vi "UHR-Fleezers Control (host) - 12.8.vi"() -> ()   [LabVIEW 2012] (continued)
        "Time/f+b scan (s) (MCL)" <- w1868
        n1295 = Divide(x=w1894, y=w1874) -> (x/y=→"N sets should be saved (MCL)":dbl)
        n1296 = Multiply(x=w1868, y=w1867) -> (x*y=→"Total Time (s)":dbl)
        n1297 = Not(x="Fast Scan Dir") -> (.not. x?=w1872:bool)
        n1298 = xnode "Read/Write Control"("FPGA VI Reference In"=w1860, "Scan steps (MCL)"="Scan steps (MCL)", "Number of scans (MCL)"=w1867, "Cycles per step (MCL)"=w1885, "Scan freq.  increment (MCL)"=w1865, "1D or 2D Scan?"="2D or 1D Scan", "MCL Scan Axis"=w1872, "Cont. Scan (MCL)"="Continuous MCL Scanning") -> ("error out"=w1896:errorcluster)  [unwired: 1 in, 1 out]
      }
      event "Read Cal": Value Change {
        w1898 = 1000.0 ("y")
        n1299 = event-data() -> ()  [unwired: 7 out]
        n1300 = local read "Save file name"() -> (w1923:path)
        n1301 = local write "Read Cal"(FALSE ("Read Cal")) -> ()
        n1302 = Strip Path(path=w1923) -> (stripped path=w1922:path)  [unwired: 1 out]
        n1303 = Path To String(path=w1922) -> (string=w1921:string)
        n1304 = Concatenate Strings(w1921, "\\current.cal" ("string")) -> (w1919:string)
        n1305 = String To Path(string=w1919) -> (path=w1918:path)
        n1306 = Open/Create/Replace File(file path (use dialog)=w1918, operation (0:open)=T29."open", access (0:read/write)=enum16{"read/write", "read-only", "write-only"}."read-only") -> (refnum out=w1926:refnum<file>, error out=w1912:errorcluster)  [unwired: 1 in, 3 out]
        n1307 = Deny Access(4:w1912, 7:w1926) -> (0:w1911:errorcluster, 3:w1917:refnum<file>)  [unwired: 1 out]
        n1308 = Read from Binary File(5:0.0, 8:w1911, 9:T28."big-endian, network order" ("byte order (0:big-endian, network order)"), 10:-1 ("count (1)"), 11:w1917) -> (0:w1910:errorcluster, 2:w1908:dbl[], 3:w1913:refnum<file>)  [unwired: 2 out]
        n1309 = Array To Cluster(array=w1908) -> (cluster=w1907:T31)
        n1310 = Unbundle(w1907) -> ("[0]"=w1906:dbl, "[1]"=w1905:dbl, "[2]"=w1904:dbl, "[3]"=w1903:dbl, "[4]"=w1902:dbl, "[5]"=w1901:dbl)
        n1311 = Close File(refnum=w1913, error in=w1910) -> (error out=→"Read cal error":errorcluster)  [unwired: 1 out]
        n1312 = Multiply(x=w1901, y=w1898) -> (x*y=w1899:dbl)
        n1313 = local write "T2 kappa_x (pN/nm)"(w1903) -> ()
        n1314 = local write "T1 kappa_x (pN/nm)"(w1904) -> ()
        n1315 = local write "T1 alpha_x (nm/V)"(w1906) -> ()
        n1316 = local write "T2 alpha_x (nm/V)"(w1905) -> ()
        n1317 = Multiply(x=w1902, y=w1898) -> (x*y=w1900:dbl)
        n1318 = local write "T1 offset_x (mV)"(w1900) -> ()
        n1319 = local write "T2 offset_x (mV)"(w1899) -> ()
      }
      event "Abort MCL Scan": Value Change {
        n1320 = event-data() -> ()  [unwired: 7 out]
        n1321 = local write "MCL Scanning"(FALSE ("MCL Scanning")) -> ()
        n1322 = xnode "Read/Write Control"("FPGA VI Reference In"=w1927, "Abort scan (MCL)"="Abort MCL Scan") -> ("error out"=w1930:errorcluster)  [unwired: 1 in, 1 out]
      }
      event "Update Count (MCL)": Value Change {
        n1323 = event-data() -> ()  [unwired: 7 out]
        n1324 = xnode "Read/Write Control"("FPGA VI Reference In"=w1931, "MCL count"="Update Count (MCL)") -> ("error out"=w1933:errorcluster)  [unwired: 1 in, 1 out]
      }
      event "+ phase (MCL)", "- phase (MCL)": Value Change {
        n1325 = event-data() -> ()  [unwired: 7 out]
        n1326 = Or(x="- phase (MCL)", y="+ phase (MCL)") -> (x .or. y?=w1937:bool)
        n1327 = Negate(x="Phase adjust (MCL)") -> (-x=w1943:i16)
        n1328 = Select(t=w1943, s="+ phase (MCL)", f="Phase adjust (MCL)") -> (s? t:f=w1941:i16)
        n1329 = xnode "Read/Write Control"("FPGA VI Reference In"=w1934, "Phase count adjustment (MCL)"=w1941) -> ("FPGA VI Reference Out"=w1938:T20, "error out"=w1939:errorcluster)  [unwired: 1 in]
        n1330 = xnode "Read/Write Control"("FPGA VI Reference In"=w1938, "error in"=w1939, "+ phase (MCL)"=w1937) -> ("error out"=w1936:errorcluster)  [unwired: 1 out]
      }
      event "Abort AOD Scan": Value Change {
        n1331 = event-data() -> ()  [unwired: 7 out]
        n1332 = xnode "Read/Write Control"("FPGA VI Reference In"=w1944, "Abort scan"="Abort AOD Scan") -> ("error out"=w1946:errorcluster)  [unwired: 1 in, 1 out]
      }
      event "Continuous AOD Scanning": Value Change {
        n1333 = event-data() -> ()  [unwired: 7 out]
        n1334 = xnode "Read/Write Control"("FPGA VI Reference In"=w1947, "Cont. Scan"="Continuous AOD Scanning") -> ("error out"=w1949:errorcluster)  [unwired: 1 in, 1 out]
      }
      event "Index": Value Change {
        n1335 = event-data() -> ()  [unwired: 7 out]
        n1336 = call "Create new save file.vi"("Insert"="", "Ext"=".dat" ("string"), "Index In"="Index") -> ("Path Out"=→"Save file name":path, "Index Out"=w1950:dbl)
        "Save index" <- w1950
        n1337 = local write "Index"(w1950) -> ()
      }
      event "AO1", "AO2": Value Change {
        w1964 = 10.0 ("y")
        w1963 = 32767.0 ("y")
        n1338 = event-data() -> ()  [unwired: 7 out]
        n1339 = local read "AO2"() -> (w1962:dbl)
        n1340 = local read "AO1"() -> (w1959:dbl)
        n1341 = Multiply(x=w1959, y=w1963) -> (x*y=w1958:dbl)
        n1342 = Multiply(x=w1962, y=w1963) -> (x*y=w1961:dbl)
        n1343 = Divide(x=w1958, y=w1964) -> (x/y=w1957:dbl)
        n1344 = Divide(x=w1961, y=w1964) -> (x/y=w1960:dbl)
        n1345 = To Word Integer(number=w1957) -> (16bit integer=w1965:i16)
        n1346 = To Word Integer(number=w1960) -> (16bit integer=w1966:i16)
        n1347 = xnode "Read/Write Control"("FPGA VI Reference In"=w1955, "AO1"=w1965, "AO2"=w1966) -> ("error out"=w1956:errorcluster)  [unwired: 1 in, 1 out]
      }
      event "Inject Pump 1": Value Change {
        n1348 = event-data() -> ()  [unwired: 7 out]
        n1349 = local read "Use Harvard pumps\nfor beads (else Chemyx)"() -> (w1968:bool)
        n1350 = case shown="True" w1968 {
          tunnel: "Inject Pump 1" -> [w1972 w2010]
          tunnel: w1967 -> [_ w2011]
          frame False {
            n1351 = local read "Pump write delay (ms)"() -> (w1971:dbl)
            n1352 = local read "Chemyx Syringe Pump Serial Port"() -> (w1970:refnum<visa-resource-name>)
            n1353 = case shown="True" w1972 {
              tunnel: w1971 -> [w1978 w1992]
              tunnel: w1970 -> [w1975 w1991]
              frame False {
                n1354 = flat-sequence {
                  tunnel: w1975 -> [w1979]
                  tunnel: [w1979] -> w1976
                  tunnel: w1978 -> [_]
                  tunnel: [w1982] -> w1977
                  tunnel: w1976 -> [w1982]
                  tunnel: w1977 -> [w1983]
                  tunnel: [w1983] -> w1973
                  tunnel: [w1985] -> w1974
                  tunnel: w1973 -> [w1985]
                  tunnel: w1974 -> [w1987]
                  frame #0 {
                    n1355 = call "Write to pump.vi"("string"="enter pump1", "VISA resource name"=w1979) -> ()  [unwired: 1 out]
                  }
                  frame #1 {
                    n1356 = Wait (ms)(milliseconds to wait="Pump pause delay (ms)") -> ()  [unwired: 1 out]
                  }
                  frame #2 {
                    n1357 = call "Write to pump.vi"("string"="stop", "VISA resource name"=w1983) -> ()  [unwired: 1 out]
                  }
                  frame #3 {
                    n1358 = Wait (ms)(milliseconds to wait=u32 500) -> ()  [unwired: 1 out]
                  }
                  frame #4 {
                    n1359 = call "Write to pump.vi"("string"="stop", "VISA resource name"=w1987) -> ()  [unwired: 1 out]
                  }
                }
              }
              frame True {
                n1360 = flat-sequence {
                  tunnel: w1991 -> [w2001]
                  tunnel: w1992 -> [w1996]
                  tunnel: w1992 -> [w2003]
                  tunnel: w1991 -> [w2004]
                  tunnel: [w2004] -> w1989
                  tunnel: [w2006] -> w1990
                  tunnel: w1989 -> [w2006]
                  tunnel: w1990 -> [w2008]
                  frame #0 {
                    n1361 = local read "All Pump Parameters"() -> (w1995:T5)
                    n1362 = Unbundle By Name(w1995) -> ("Pump 1"=w2002:T32)
                    n1363 = call "Set pump parameters.vi"("Pump write delay (ms)"=w1996, "Volume (uL)"="Ch 1 Inject Volume (uL)", "Rate (uL/h)"="Ch 1 Inject Rate (ul/h)", "Units"=4.0, "Pump #"=1.0, "Pump Parameters In"=w2002, "VISA resource name"=w2001) -> ("Pump Parameters Out"=w1994:T32)  [unwired: 3 in]
                    n1364 = Bundle By Name(cluster=w1995, "Pump 1"=w1994) -> (w1993:T5)
                    n1365 = local write "All Pump Parameters"(w1993) -> ()
                  }
                  frame #1 {
                    n1366 = Wait (ms)(milliseconds to wait=w2003) -> ()  [unwired: 1 out]
                  }
                  frame #2 {
                    n1367 = call "Write to pump.vi"("string"="start", "VISA resource name"=w2004) -> ()  [unwired: 1 out]
                  }
                  frame #3 {
                    n1368 = Wait (ms)(milliseconds to wait=u32 500) -> ()  [unwired: 1 out]
                  }
                  frame #4 {
                    n1369 = call "Write to pump.vi"("string"="start", "VISA resource name"=w2008) -> ()  [unwired: 1 out]
                  }
                }
              }
            }
          }
          frame True {
            n1370 = case shown="False" w2010 {
              tunnel: w2011 -> [w2012 w2022]
              frame False {
                n1371 = flat-sequence {
                  tunnel: w2012 -> [w2014]
                  frame #0 {
                    n1372 = local write "Flushing P1"(FALSE ("Flushing P1")) -> ()
                    n1373 = Concatenate Strings("stop" ("string"), "\r") -> (w2016:string)
                    n1374 = VISA Write(VISA resource name=w2014, write buffer=w2016) -> ()  [unwired: 1 in, 3 out]
                  }
                  frame #1 {
                    n1375 = property on="Clear Volume P1" class="Bool (strict)"("Val(Sgnl)"=TRUE ("Value (Signaling)")) -> ()  [unwired: 2 in, 2 out]
                  }
                }
              }
              frame True {
                n1376 = local read "Normal Flow Rate (ul/h) P1"() -> (w2020:dbl)
                n1377 = Number To Decimal String(number=w2020) -> (decimal integer string=w2026:string)  [unwired: 1 in]
                n1378 = Concatenate Strings("irate  " ("string"), w2026, " u/h" ("string"), "\r") -> (w2024:string)
                n1379 = VISA Write(VISA resource name=w2022, write buffer=w2024) -> (VISA resource name out=w2021:refnum<visa-resource-name>)  [unwired: 1 in, 2 out]
                n1380 = Concatenate Strings("irun" ("string"), "\r") -> (w2028:string)
                n1381 = VISA Write(VISA resource name=w2021, write buffer=w2028) -> ()  [unwired: 1 in, 3 out]
              }
            }
          }
        }
      }
      event "Inject Pump 3": Value Change {
        n1382 = event-data() -> ()  [unwired: 7 out]
        n1383 = local read "Use Harvard pumps\nfor beads (else Chemyx)"() -> (w2031:bool)
        n1384 = case shown="True" w2031 {
          tunnel: "Inject Pump 3" -> [w2035 w2074]
          tunnel: w2030 -> [_ w2073]
          frame False {
            n1385 = local read "Pump write delay (ms)"() -> (w2034:dbl)
            n1386 = case shown="True" w2035 {
              tunnel: w2034 -> [w2041 w2055]
              tunnel: "Chemyx Syringe Pump Serial Port" -> [w2038 w2054]
              frame False {
                n1387 = flat-sequence {
                  tunnel: w2038 -> [w2042]
                  tunnel: [w2042] -> w2039
                  tunnel: w2041 -> [_]
                  tunnel: [w2045] -> w2040
                  tunnel: w2039 -> [w2045]
                  tunnel: w2040 -> [w2046]
                  tunnel: [w2046] -> w2036
                  tunnel: [w2048] -> w2037
                  tunnel: w2036 -> [w2048]
                  tunnel: w2037 -> [w2050]
                  frame #0 {
                    n1388 = call "Write to pump.vi"("string"="enter pump3", "VISA resource name"=w2042) -> ()  [unwired: 1 out]
                  }
                  frame #1 {
                    n1389 = local read "Pump pause delay (ms)"() -> (w2044:u32)
                    n1390 = Wait (ms)(milliseconds to wait=w2044) -> ()  [unwired: 1 out]
                  }
                  frame #2 {
                    n1391 = call "Write to pump.vi"("string"="stop", "VISA resource name"=w2046) -> ()  [unwired: 1 out]
                  }
                  frame #3 {
                    n1392 = Wait (ms)(milliseconds to wait=u32 0) -> ()  [unwired: 1 out]
                  }
                  frame #4 {
                    n1393 = call "Write to pump.vi"("string"="stop", "VISA resource name"=w2050) -> ()  [unwired: 1 out]
                  }
                }
              }
              frame True {
                n1394 = flat-sequence {
                  tunnel: w2054 -> [w2064]
                  tunnel: w2055 -> [w2059]
                  tunnel: w2055 -> [w2066]
                  tunnel: w2054 -> [w2067]
                  tunnel: [w2067] -> w2053
                  tunnel: [w2070] -> w2052
                  tunnel: w2053 -> [w2070]
                  tunnel: w2052 -> [w2071]
                  frame #0 {
                    n1395 = local read "All Pump Parameters"() -> (w2058:T5)
                    n1396 = Unbundle By Name(w2058) -> ("Pump 3"=w2065:T32)
                    n1397 = call "Set pump parameters.vi"("Pump write delay (ms)"=w2059, "Volume (uL)"="Ch 3 Inject Volume (uL)", "Rate (uL/h)"="Ch 3 Inject Rate (ul/h)", "Units"=4.0, "Pump #"=3.0, "Pump Parameters In"=w2065, "VISA resource name"=w2064) -> ("Pump Parameters Out"=w2057:T32)  [unwired: 3 in]
                    n1398 = Bundle By Name(cluster=w2058, "Pump 3"=w2057) -> (w2056:T5)
                    n1399 = local write "All Pump Parameters"(w2056) -> ()
                  }
                  frame #1 {
                    n1400 = Wait (ms)(milliseconds to wait=w2066) -> ()  [unwired: 1 out]
                  }
                  frame #2 {
                    n1401 = call "Write to pump.vi"("string"="start", "VISA resource name"=w2067) -> ()  [unwired: 1 out]
                  }
                  frame #3 {
                    n1402 = Wait (ms)(milliseconds to wait=u32 500) -> ()  [unwired: 1 out]
                  }
                  frame #4 {
                    n1403 = call "Write to pump.vi"("string"="start", "VISA resource name"=w2071) -> ()  [unwired: 1 out]
                  }
                }
              }
            }
          }
          frame True {
            n1404 = case shown="False" w2074 {
              tunnel: w2073 -> [w2075 w2082]
              frame False {
                n1405 = flat-sequence {
                  tunnel: w2075 -> [w2077]
                  frame #0 {
                    n1406 = local write "Flushing P3"(FALSE ("Flushing P3")) -> ()
                    n1407 = Concatenate Strings("stop" ("string"), "\r") -> (w2079:string)
                    n1408 = VISA Write(VISA resource name=w2077, write buffer=w2079) -> ()  [unwired: 1 in, 3 out]
                  }
                  frame #1 {
                    n1409 = property on="Clear Volume P3" class="Bool (strict)"("Val(Sgnl)"=TRUE ("Value (Signaling)")) -> ()  [unwired: 2 in, 2 out]
                  }
                }
              }
              frame True {
                n1410 = local read "Normal Flow Rate (ul/h) P3"() -> (w2083:dbl)
                n1411 = Number To Decimal String(number=w2083) -> (decimal integer string=w2089:string)  [unwired: 1 in]
                n1412 = Concatenate Strings("irate  " ("string"), w2089, " u/h" ("string"), "\r") -> (w2087:string)
                n1413 = VISA Write(VISA resource name=w2082, write buffer=w2087) -> (VISA resource name out=w2085:refnum<visa-resource-name>)  [unwired: 1 in, 2 out]
                n1414 = Concatenate Strings("irun" ("string"), "\r") -> (w2091:string)
                n1415 = VISA Write(VISA resource name=w2085, write buffer=w2091) -> ()  [unwired: 1 in, 3 out]
              }
            }
          }
        }
      }
      event "Inject Pump 2": Value Change {
        n1416 = event-data() -> ()  [unwired: 7 out]
        n1417 = local read "Pump write delay (ms)"() -> (w2095:dbl)
        n1418 = flat-sequence {
          tunnel: w2093 -> [w2108]
          tunnel: w2095 -> [w2104]
          tunnel: "Inject Pump 2" -> [_]
          tunnel: w2095 -> [w2110]
          tunnel: w2093 -> [w2111]
          frame #0 {
            n1419 = local read "All Pump Parameters"() -> (w2103:T5)
            n1420 = Multiply(x=60.0, y="Flush Center Ch Rate (ul/m)") -> (x*y=w2100:dbl)
            n1421 = Unbundle By Name(w2103) -> ("Pump 2"=w2109:T32)
            n1422 = call "Set pump parameters.vi"("Pump write delay (ms)"=w2104, "Volume (uL)"="Flush Center Ch Volume (uL)", "Rate (uL/h)"=w2100, "Units"=3.0, "Pump #"=2.0, "Pump Parameters In"=w2109, "VISA resource name"=w2108) -> ("Pump Parameters Out"=w2102:T32)  [unwired: 3 in]
            n1423 = Bundle By Name(cluster=w2103, "Pump 2"=w2102) -> (w2101:T5)
            n1424 = local write "All Pump Parameters"(w2101) -> ()
            n1425 = Add(x="Flush Center Ch Volume (uL)", y="Total Volume\nFlushed (uL)") -> (x+y=w2097:dbl)
            n1426 = local write "Total Volume\nFlushed (uL)"(w2097) -> ()
          }
          frame #1 {
            n1427 = Wait (ms)(milliseconds to wait=w2110) -> ()  [unwired: 1 out]
          }
          frame #2 {
            n1428 = call "Write to pump.vi"("string"="start", "VISA resource name"=w2111) -> ()  [unwired: 1 out]
          }
        }
        n1429 = local read "Chemyx Syringe Pump Serial Port"() -> (w2093:refnum<visa-resource-name>)
      }
      event "Sample Channel\nFlow": Value Change {
        n1430 = event-data() -> ()  [unwired: 7 out]
        n1431 = Select(t="irun" ("string"), s="Sample Channel\nFlow", f="stop" ("string")) -> (s? t:f=w2115:string)
        n1432 = Concatenate Strings(w2115, "\r") -> (w2118:string)
        n1433 = VISA Write(VISA resource name=w2113, write buffer=w2118) -> ()  [unwired: 1 in, 3 out]
      }
      event "Start Flow": Value Change {
        n1434 = event-data() -> ()  [unwired: 7 out]
        n1435 = local write "Sample Channel\nFlow"(TRUE ("Sample Channel\nFlow")) -> ()
        n1436 = local write "Start Flow"(FALSE ("Start Flow")) -> ()
        n1437 = Concatenate Strings("irun" ("string"), "\r") -> (w2124:string)
        n1438 = VISA Write(VISA resource name=w2120, write buffer=w2124) -> ()  [unwired: 1 in, 3 out]
      }
      event "Stop Flow": Value Change {
        w2126 = FALSE ("Stop Flow")
        n1439 = event-data() -> ()  [unwired: 7 out]
        n1440 = local write "Stop Flow"(w2126) -> ()
        n1441 = local write "Sample Channel\nFlow"(w2126) -> ()
        n1442 = Concatenate Strings("stop" ("string"), "\r") -> (w2129:string)
        n1443 = VISA Write(VISA resource name=w2127, write buffer=w2129) -> ()  [unwired: 1 in, 3 out]
      }
      event "Flow rate (uL/h)": Value Change {
        n1444 = event-data() -> ()  [unwired: 7 out]
        n1445 = Number To Decimal String(number="Flow rate (uL/h)") -> (decimal integer string=w2136:string)  [unwired: 1 in]
        n1446 = Concatenate Strings("irate  " ("string"), w2136, " u/h" ("string"), "\r") -> (w2135:string)
        n1447 = VISA Write(VISA resource name=w2132, write buffer=w2135) -> ()  [unwired: 1 in, 3 out]
      }
      event "Flush Sample": Value Change {
        n1448 = event-data() -> ()  [unwired: 7 out]
        n1449 = flat-sequence {
          tunnel: w2141 -> [w2169]
          tunnel: [w2149] -> w2140
          tunnel: [w2143] -> w2138
          tunnel: w2140 -> [w2173]
          tunnel: [w2173] -> w2139
          tunnel: w2138 -> [w2172]
          tunnel: w2139 -> [w2178]
          frame #0 {
            # "set paramaters (rate, volume) for flush, clear volume"
            n1450 = Number To Decimal String(number="Flush rate (uL/m)") -> (decimal integer string=w2165:string)  [unwired: 1 in]
            n1451 = Concatenate Strings("irate  " ("string"), w2165, " u/m" ("string"), "\r") -> (w2167:string)
            n1452 = VISA Write(VISA resource name=w2169, write buffer=w2167) -> (VISA resource name out=w2163:refnum<visa-resource-name>)  [unwired: 1 in, 2 out]
            n1453 = Reciprocal(x="Flush rate (uL/m)") -> (1/x=w2146:dbl)
            n1454 = Number To Decimal String(number="Volume (uL)") -> (decimal integer string=w2154:string)  [unwired: 1 in]
            n1455 = Multiply(x="Volume (uL)", y=w2146) -> (x*y=w2145:dbl)
            n1456 = Concatenate Strings("tvolume  " ("string"), w2154, " u" ("string"), "\r") -> (w2152:string)
            n1457 = Multiply(x=w2145, y=60000.0) -> (x*y=w2143:dbl)
            n1458 = VISA Write(VISA resource name=w2163, write buffer=w2152) -> (VISA resource name out=w2151:refnum<visa-resource-name>)  [unwired: 1 in, 2 out]
            n1459 = Concatenate Strings("cvolume" ("string"), "\r") -> (w2150:string)
            n1460 = VISA Write(VISA resource name=w2151, write buffer=w2150) -> (VISA resource name out=w2161:refnum<visa-resource-name>)  [unwired: 1 in, 2 out]
            n1461 = Concatenate Strings("irun" ("string"), "\r") -> (w2159:string)
            n1462 = VISA Write(VISA resource name=w2161, write buffer=w2159) -> (VISA resource name out=w2149:refnum<visa-resource-name>)  [unwired: 1 in, 2 out]
          }
          frame #1 {
            # "Have to wait until\nflow is done to reset\nrate"
            n1463 = Add(x=w2172, y=100.0) -> (x+y=w2171:dbl)
            n1464 = Wait (ms)(milliseconds to wait=w2171) -> ()  [unwired: 1 out]
          }
          frame #2 {
            # "reset flow rate to usual flow rate"
            n1465 = local read "Flow rate (uL/h)"() -> (w2184:dbl)
            n1466 = Number To Decimal String(number=w2184) -> (decimal integer string=w2182:string)  [unwired: 1 in]
            n1467 = Concatenate Strings("irate  " ("string"), w2182, " u/h" ("string"), "\r") -> (w2180:string)
            n1468 = VISA Write(VISA resource name=w2178, write buffer=w2180) -> (VISA resource name out=w2174:refnum<visa-resource-name>)  [unwired: 1 in, 2 out]
            n1469 = Concatenate Strings("cvolume" ("string"), "\r") -> (w2175:string)
            n1470 = VISA Write(VISA resource name=w2174, write buffer=w2175) -> ()  [unwired: 1 in, 3 out]
          }
        }
      }
      event "Flush Pump 3": Value Change {
        n1471 = event-data() -> ()  [unwired: 7 out]
        n1472 = flat-sequence {
          tunnel: w2185 -> [w2188]
          frame #0 {
            # "set paramaters (rate, volume) for flush, clear volume"
            n1473 = Number To Decimal String(number="Flush rate (uL/m) P3") -> (decimal integer string=w2210:string)  [unwired: 1 in]
            n1474 = local write "Inject Pump 3"(TRUE ("Inject Pump 3")) -> ()
            n1475 = Concatenate Strings("irate  " ("string"), w2210, " u/m" ("string"), "\r") -> (w2212:string)
            n1476 = VISA Write(VISA resource name=w2188, write buffer=w2212) -> (VISA resource name out=w2208:refnum<visa-resource-name>)  [unwired: 1 in, 2 out]
            n1477 = Reciprocal(x="Flush rate (uL/m) P3") -> (1/x=w2192:dbl)
            n1478 = Number To Decimal String(number="Volume (uL) P3") -> (decimal integer string=w2199:string)  [unwired: 1 in]
            n1479 = Multiply(x="Volume (uL) P3", y=w2192) -> (x*y=w2191:dbl)
            n1480 = Concatenate Strings("tvolume  " ("string"), w2199, " u" ("string"), "\r") -> (w2197:string)
            n1481 = Multiply(x=w2191, y=60.0) -> (x*y=→"HP3 Flush Time (s)":dbl)
            n1482 = VISA Write(VISA resource name=w2208, write buffer=w2197) -> (VISA resource name out=w2196:refnum<visa-resource-name>)  [unwired: 1 in, 2 out]
            n1483 = Concatenate Strings("cvolume" ("string"), "\r") -> (w2195:string)
            n1484 = VISA Write(VISA resource name=w2196, write buffer=w2195) -> (VISA resource name out=w2206:refnum<visa-resource-name>)  [unwired: 1 in, 2 out]
            n1485 = Concatenate Strings("irun" ("string"), "\r") -> (w2204:string)
            n1486 = VISA Write(VISA resource name=w2206, write buffer=w2204) -> ()  [unwired: 1 in, 3 out]
          }
          frame #1 {
            "Flushing P3" <- TRUE ("Flushing P3")
          }
        }
      }
      event "Flush Pump 1": Value Change {
        n1487 = event-data() -> ()  [unwired: 7 out]
        n1488 = flat-sequence {
          tunnel: [w2226] -> w2216
          tunnel: w2215 -> [w2219]
          tunnel: w2216 -> [_]
          frame #0 {
            # "set paramaters (rate, volume) for flush, clear volume"
            n1489 = local write "Inject Pump 1"(TRUE ("Inject Pump 1")) -> ()
            n1490 = Number To Decimal String(number="Flush rate (uL/m) P1") -> (decimal integer string=w2242:string)  [unwired: 1 in]
            n1491 = Concatenate Strings("irate  " ("string"), w2242, " u/m" ("string"), "\r") -> (w2244:string)
            n1492 = VISA Write(VISA resource name=w2219, write buffer=w2244) -> (VISA resource name out=w2240:refnum<visa-resource-name>)  [unwired: 1 in, 2 out]
            n1493 = Reciprocal(x="Flush rate (uL/m) P1") -> (1/x=w2223:dbl)
            n1494 = Number To Decimal String(number="Volume (uL) P1") -> (decimal integer string=w2231:string)  [unwired: 1 in]
            n1495 = Multiply(x="Volume (uL) P1", y=w2223) -> (x*y=w2222:dbl)
            n1496 = Concatenate Strings("tvolume  " ("string"), w2231, " u" ("string"), "\r") -> (w2229:string)
            n1497 = Multiply(x=w2222, y=60.0) -> (x*y=→"HP1 Flush Time (s)":dbl)
            n1498 = VISA Write(VISA resource name=w2240, write buffer=w2229) -> (VISA resource name out=w2228:refnum<visa-resource-name>)  [unwired: 1 in, 2 out]
            n1499 = Concatenate Strings("cvolume" ("string"), "\r") -> (w2227:string)
            n1500 = VISA Write(VISA resource name=w2228, write buffer=w2227) -> (VISA resource name out=w2238:refnum<visa-resource-name>)  [unwired: 1 in, 2 out]
            n1501 = Concatenate Strings("irun" ("string"), "\r") -> (w2236:string)
            n1502 = VISA Write(VISA resource name=w2238, write buffer=w2236) -> (VISA resource name out=w2226:refnum<visa-resource-name>)  [unwired: 1 in, 2 out]
          }
          frame #1 {
            "Flushing P1" <- TRUE ("Flushing P3")
          }
        }
      }
      event "Clear Volume": Value Change {
        n1503 = event-data() -> ()  [unwired: 7 out]
        n1504 = Concatenate Strings("cvolume" ("string"), "\r") -> (w2248:string)
        n1505 = VISA Write(VISA resource name=w2247, write buffer=w2248) -> ()  [unwired: 1 in, 3 out]
      }
      event "Clear Volume P3": Value Change {
        n1506 = event-data() -> ()  [unwired: 7 out]
        n1507 = Concatenate Strings("cvolume" ("string"), "\r") -> (w2254:string)
        n1508 = VISA Write(VISA resource name=w2253, write buffer=w2254) -> ()  [unwired: 1 in, 3 out]
        n1509 = local write "Clear Volume P3"(FALSE ("Clear Volume P3")) -> ()
      }
      event "Clear Volume P1": Value Change {
        n1510 = event-data() -> ()  [unwired: 7 out]
        n1511 = Concatenate Strings("cvolume" ("string"), "\r") -> (w2259:string)
        n1512 = local write "Clear Volume P1"(FALSE ("Clear Volume P1")) -> ()
        n1513 = VISA Write(VISA resource name=w2258, write buffer=w2259) -> ()  [unwired: 1 in, 3 out]
      }
      event "Display On P3": Value Change {
        n1514 = event-data() -> ()  [unwired: 7 out]
        n1515 = Select(t="dim 100", s="Display On P3", f="dim 0") -> (s? t:f=w2265:string)
        n1516 = Concatenate Strings(w2265, "\r") -> (w2267:string)
        n1517 = VISA Write(VISA resource name=w2262, write buffer=w2267) -> ()  [unwired: 1 in, 3 out]
      }
      event "Display On P1": Value Change {
        n1518 = event-data() -> ()  [unwired: 7 out]
        n1519 = Select(t="dim 100", s="Display On P1", f="dim 0") -> (s? t:f=w2272:string)
        n1520 = Concatenate Strings(w2272, "\r") -> (w2274:string)
        n1521 = VISA Write(VISA resource name=w2269, write buffer=w2274) -> ()  [unwired: 1 in, 3 out]
      }
      event "Retract Pump 3": Value Change {
        n1522 = event-data() -> ()  [unwired: 7 out]
        n1523 = local write "Retract Pump 3"(FALSE ("Retract Pump 3")) -> ()
        n1524 = case shown="True" "Retract Pump 3" {
          tunnel: w2276 -> [_ w2279]
          frame False {
          }
          frame True {
            n1525 = Number To Decimal String(number="Retract Rate (uL/m)") -> (decimal integer string=w2297:string)  [unwired: 1 in]
            n1526 = Concatenate Strings("wrate  " ("string"), w2297, " u/m" ("string"), "\r") -> (w2299:string)
            n1527 = VISA Write(VISA resource name=w2279, write buffer=w2299) -> (VISA resource name out=w2290:refnum<visa-resource-name>)  [unwired: 1 in, 2 out]
            n1528 = Number To Decimal String(number="Retract Vol 3 (uL)") -> (decimal integer string=w2292:string)  [unwired: 1 in]
            n1529 = Concatenate Strings("tvolume  " ("string"), w2292, " u" ("string"), "\r") -> (w2289:string)
            n1530 = VISA Write(VISA resource name=w2290, write buffer=w2289) -> (VISA resource name out=w2285:refnum<visa-resource-name>)  [unwired: 1 in, 2 out]
            n1531 = Concatenate Strings("cvolume" ("string"), "\r") -> (w2286:string)
            n1532 = VISA Write(VISA resource name=w2285, write buffer=w2286) -> (VISA resource name out=w2280:refnum<visa-resource-name>)  [unwired: 1 in, 2 out]
            n1533 = Concatenate Strings("wrun" ("string"), "\r") -> (w2281:string)
            n1534 = VISA Write(VISA resource name=w2280, write buffer=w2281) -> ()  [unwired: 1 in, 3 out]
          }
        }
      }
      event "Retract Pump 1": Value Change {
        n1535 = event-data() -> ()  [unwired: 7 out]
        n1536 = local write "Retract Pump 1"(FALSE ("Retract Pump 1")) -> ()
        n1537 = case shown="True" "Retract Pump 1" {
          tunnel: w2301 -> [_ w2306]
          frame False {
          }
          frame True {
            n1538 = local read "Retract Rate (uL/m)"() -> (w2304:dbl)
            n1539 = Number To Decimal String(number=w2304) -> (decimal integer string=w2322:string)  [unwired: 1 in]
            n1540 = Concatenate Strings("wrate  " ("string"), w2322, " u/m" ("string"), "\r") -> (w2324:string)
            n1541 = VISA Write(VISA resource name=w2306, write buffer=w2324) -> (VISA resource name out=w2316:refnum<visa-resource-name>)  [unwired: 1 in, 2 out]
            n1542 = Number To Decimal String(number="Retract Vol 1 (uL)") -> (decimal integer string=w2318:string)  [unwired: 1 in]
            n1543 = Concatenate Strings("tvolume  " ("string"), w2318, " u" ("string"), "\r") -> (w2315:string)
            n1544 = VISA Write(VISA resource name=w2316, write buffer=w2315) -> (VISA resource name out=w2312:refnum<visa-resource-name>)  [unwired: 1 in, 2 out]
            n1545 = Concatenate Strings("cvolume" ("string"), "\r") -> (w2313:string)
            n1546 = VISA Write(VISA resource name=w2312, write buffer=w2313) -> (VISA resource name out=w2307:refnum<visa-resource-name>)  [unwired: 1 in, 2 out]
            n1547 = Concatenate Strings("wrun" ("string"), "\r") -> (w2308:string)
            n1548 = VISA Write(VISA resource name=w2307, write buffer=w2308) -> ()  [unwired: 1 in, 3 out]
          }
        }
      }
      event "Flip Green Filter": Value Change {
        n1549 = event-data() -> ()  [unwired: 7 out]
        n1550 = Not(x="Flip Green Filter") -> (.not. x?=w2327:bool)
        n1551 = local write "Flip Green Filter"(w2327) -> ()
        n1552 = flat-sequence {
          tunnel: [w2336] -> w2332
          tunnel: [w2335] -> w2331
          tunnel: w2326 -> [w2334]
          tunnel: [w2339] -> w2330
          tunnel: w2332 -> [w2339]
          tunnel: [w2338] -> w2329
          tunnel: w2331 -> [w2338]
          tunnel: w2330 -> [w2343]
          tunnel: w2329 -> [w2342]
          tunnel: [w2341] -> w2333
          frame #0 {
            n1553 = xnode "Read/Write Control"("FPGA VI Reference In"=w2334, "Green Filter Flipper"=TRUE) -> ("FPGA VI Reference Out"=w2336:T20, "error out"=w2335:errorcluster)  [unwired: 1 in]
          }
          frame #1 {
            n1554 = Wait (ms)(milliseconds to wait=u32 100) -> ()  [unwired: 1 out]
          }
          frame #2 {
            n1555 = xnode "Read/Write Control"("FPGA VI Reference In"=w2343, "error in"=w2342, "Green Filter Flipper"=FALSE) -> ("error out"=w2341:errorcluster)  [unwired: 1 out]
          }
        }
      }
      event "Pump 1 contents", "Pump 3 contents": Value Change {
        n1556 = event-data() -> ()  [unwired: 7 out]
        n1557 = local read "Pump 1 contents"() -> (→"Pump 1 cont disp":string)
        n1558 = local read "Pump 3 contents"() -> (→"Pump 3 cont disp":string)
      }
      event "Reset Trap Pos. FB": Value Change {
        n1559 = event-data() -> ()  [unwired: 7 out]
        n1560 = xnode "Read/Write Control"("FPGA VI Reference In"=w2347, "Trap Pos. FB Reset"="Reset Trap Pos. FB") -> ()  [unwired: 1 in, 2 out]
      }
      event "Rem fb disp offset": Value Change {
        n1561 = event-data() -> ()  [unwired: 7 out]
        n1562 = local write "Rem fb disp offset"(FALSE ("Rem fb disp offset")) -> ()
        n1563 = local read "Mean T1 Position (nm)"() -> (w2350:dbl)
        n1564 = local read "FB Trap Pos Offset"() -> (w2351:dbl)
        n1565 = Subtract(x=w2351, y=w2350) -> (x-y=w2349:dbl)
        n1566 = local write "FB Trap Pos Offset"(w2349) -> ()
      }
      event "Threshold (nm)": Value Change {
        n1567 = event-data() -> ()  [unwired: 7 out]
        n1568 = flat-sequence {
          tunnel: [w2356] -> w2354
          tunnel: w2353 -> [w2355]
          tunnel: w2354 -> [w2367]
          frame #0 {
            n1569 = xnode "Read/Write Control"("FPGA VI Reference In"=w2355) -> ("FPGA VI Reference Out"=w2359:T20, "error out"=w2358:errorcluster, "FPGA TTrig Thresh"=w2360:i64)  [unwired: 1 in]
            n1570 = local read "Threshold stored (nm)"() -> (w2366:dbl)
            n1571 = local read "Threshold (nm)"() -> (w2356:dbl)
            n1572 = local read "AOM X Cal (nm/MHz)"() -> (w2364:dbl)
            n1573 = Subtract(x=w2356, y=w2366) -> (x-y=w2365:dbl)
            n1574 = Divide(x=w2365, y=w2364) -> (x/y=w2362:dbl)
            n1575 = call "IR AOM freq to word.vi"("Frequency In (MHz)"=w2362) -> ("Frequency Word Out (double)"=w2363:dbl)
            n1576 = To Quad Integer(1:w2363) -> (0:w2361:i64)
            n1577 = Add(x=w2360, y=w2361) -> (x+y=w2357:i64)
            n1578 = xnode "Read/Write Control"("FPGA VI Reference In"=w2359, "error in"=w2358, "FPGA TTrig Thresh"=w2357) -> ()  [unwired: 2 out]
          }
          frame #1 {
            "Threshold stored (nm)" <- w2367
          }
        }
      }
      event "FB Trig Integrate": Value Change {
        n1579 = event-data() -> ()  [unwired: 7 out]
        n1580 = local read "FB Trig Integrate"() -> (w2370:u32)
        n1581 = xnode "Read/Write Control"("FPGA VI Reference In"=w2368, "FB Trig Integrate"=w2370) -> ("error out"=w2369:errorcluster)  [unwired: 1 in, 1 out]
      }
      event "11": Value Change {
        n1582 = event-data() -> ()  [unwired: 7 out]
        n1583 = local read "11"() -> (w2371:bool)
        n1584 = case shown="True" w2371 {
          frame False {
          }
          frame True {
            n1585 = local read "Messages"() -> (w2373:string)
            n1586 = call "Update messages.vi"("Message to add"="You kicked it up to 11!", "Old message string"=w2373) -> ("New message string"=w2374:string)
            n1587 = call <vilib>:"Beep.vi"() -> ()  [unwired: 12 in]
            n1588 = local write "Messages"(w2374) -> ()
          }
        }
      }
      event "Trap Pos. FB ON": Value Change {
        n1589 = event-data() -> ()  [unwired: 7 out]
        n1590 = xnode "Read/Write Control"("FPGA VI Reference In"=w2375, "Force feedback"="Trap Pos. FB ON") -> ()  [unwired: 1 in, 2 out]
      }
      event "Remove Action Offset": Value Change {
        n1591 = event-data() -> ()  [unwired: 7 out]
        n1592 = local write "Remove Action Offset"(FALSE ("Remove Action Offset")) -> ()
        n1593 = local read "Trap Pos. FB Mult Factor"() -> (w2382:i64)
        n1594 = local read "Trap Pos FB Action"() -> (w2380:i64)
        n1595 = local read "Trap Pos. FB Offset Factor"() -> (w2378:i64)
        n1596 = Multiply(x=w2382, y=w2380) -> (x*y=w2381:i64)
        n1597 = Add(x=w2381, y=w2378) -> (x+y=w2379:i64)
        n1598 = local write "Trap Pos. FB Offset Factor"(w2379) -> ()
        n1599 = xnode "Read/Write Control"("FPGA VI Reference In"=w2377, "Trap Pos. FB Offset Factor"=w2379) -> ()  [unwired: 1 in, 2 out]
      }
      event "Remove Unwinding Offset": Value Change {
        n1600 = event-data() -> ()  [unwired: 7 out]
        n1601 = local write "Remove Unwinding Offset"(FALSE ("Remove Action Offset")) -> ()
        n1602 = local read "Trap Pos. FB Mult Factor"() -> (w2396:i64)
        n1603 = local read "Trap Pos FB Action"() -> (w2394:i64)
        n1604 = local read "Trap Pos. FB Offset Factor"() -> (w2393:i64)
        n1605 = Multiply(x=w2396, y=w2394) -> (x*y=w2395:i64)
        n1606 = local read "Trap Pos. FB Mult Factor"() -> (w2392:i64)
        n1607 = Add(x=w2395, y=w2393) -> (x+y=w2386:i64)
        n1608 = Multiply(x=32768, y="factor") -> (x*y=w2389:dbl)
        n1609 = Multiply(x=w2389, y=w2392) -> (x*y=w2391:dbl)
        n1610 = Subtract(x=w2386, y=w2391) -> (x-y=w2390:dbl)
        n1611 = To Quad Integer(1:w2390) -> (0:w2385:i64)
        n1612 = xnode "Read/Write Control"("FPGA VI Reference In"=w2384, "Trap Pos. FB Offset Factor"=w2385) -> ()  [unwired: 1 in, 2 out]
        n1613 = local write "Trap Pos. FB Offset Factor"(w2385) -> ()
      }
      event "Trap Pos. FB Range", "Trap Pos. FB Gains", "Trap Pos. FB Mult Factor", "Trap Pos. FB Offset Factor", "Trap Pos FB Negate Action", "Trap Pos FB Monitor\nT1 or T2", "Differential FB?", "Negate Diff?": Value Change {
        n1614 = event-data() -> ()  [unwired: 7 out]
        n1615 = Unbundle By Name("Trap Pos. FB Gains") -> ("proportional gain (Kc)"=w2401:fxp<+/-,16,8>, "integral gain (Kc*Ts/Ti)"=w2400:fxp<+/-,16,8>, "derivative gain (Kc*Td/Ts)"=w2399:fxp<+/-,16,8>)
        n1616 = local read "Negate Diff?"() -> (w2406:bool)
        n1617 = Unbundle By Name("Trap Pos. FB Range") -> ("output high"=w2404:fxp<+/-,16,1>, "output low"=w2403:fxp<+/-,16,1>)
        n1618 = xnode "Read/Write Control"("FPGA VI Reference In"=w2398, "FB2 output high"=w2404, "FB2 output low"=w2403, "P2"=w2401, "I2"=w2400, "D2"=w2399, "Trap Pos. FB Mult Factor"="Trap Pos. FB Mult Factor", "Trap Pos. FB Offset Factor"="Trap Pos. FB Offset Factor", "Trap Pos FB Negate Action"="Trap Pos FB Negate Action", "Trap Pos FB Monitor T1 or T2"="Trap Pos FB Monitor\nT1 or T2", "AI1 X Scale"="Trap Pos. AI1 X Pre-scale", "Negate Diff?"=w2406, "Diff FB Measurement?"="Differential FB?") -> ()  [unwired: 1 in, 2 out]
      }
      event "Trap Pos FB SP", "Trap Pos FB SP 2", "Use SP 2": Value Change {
        n1619 = event-data() -> ()  [unwired: 7 out]
        n1620 = Select(t="Trap Pos FB SP 2", s="Use SP 2", f="Trap Pos FB SP") -> (s? t:f=w2414:fxp<+/-,16,1>)
        n1621 = xnode "Read/Write Control"("FPGA VI Reference In"=w2413, "Trap Pos. FB SP"=w2414) -> ()  [unwired: 1 in, 2 out]
      }
      event "Offset SP2 from SP1": Value Change {
        n1622 = event-data() -> ()  [unwired: 7 out]
        n1623 = local read "Trap Pos FB SP"() -> (w2420:fxp<+/-,16,1>)
        n1624 = Add(x=w2420, y="SP2 Offset") -> (x+y=w2418:fxp<+/-,16,1>)
        n1625 = property on="Trap Pos FB SP 2" class="DigNum (strict)"("Val(Sgnl)"=w2418) -> ()  [unwired: 2 in, 2 out]
        n1626 = local write "Offset SP2 from SP1"(FALSE ("Offset SP2 from SP1")) -> ()
      }
      event "Set Reading to\nSetpoint": Value Change {
        # "This is the actual PID input signal"
        n1627 = event-data() -> ()  [unwired: 7 out]
        n1628 = local write "Set Reading to\nSetpoint"(FALSE ("Set SP to Reading")) -> ()
        n1629 = xnode "Read/Write Control"("FPGA VI Reference In"=w2422) -> ("FPGA VI Reference Out"=w2425:T20, "error out"=w2424:errorcluster, "Trap Pos FB Int-Norm Signal"=w2423:fxp<+/-,16,1>)  [unwired: 1 in]
        n1630 = local read "Differential FB?"() -> (w2426:bool)
        n1631 = case shown="False" w2426 {
          tunnel: [w2431 w2438] -> w2428
          tunnel: w2423 -> [w2429 w2438]
          frame False {
            n1632 = local read "Trap Pos FB Monitor\nT1 or T2"() -> (w2434:bool)
            n1633 = local read "Trap X AI1 (DMA)"() -> (w2437:T13)
            n1634 = Unbundle By Name(w2437) -> ("Set 1"=w2436:fxp<+/-,16,1>, "Set 2"=w2435:fxp<+/-,16,1>)
            n1635 = Select(t=w2436, s=w2434, f=w2435) -> (s? t:f=w2433:fxp<+/-,16,1>)
            n1636 = Not(x="Set SP Using...") -> (.not. x?=w2430:bool)
            n1637 = Select(t=w2429, s=w2430, f=w2433) -> (s? t:f=w2431:fxp<+/-,16,1>)
          }
          frame True {
          }
        }
        n1638 = xnode "Read/Write Control"("FPGA VI Reference In"=w2425, "error in"=w2424, "Trap Pos. FB SP"=w2428) -> ()  [unwired: 2 out]
        n1639 = local write "Trap Pos FB SP"(w2428) -> ()
      }
      event "Trap Pos. FB Out Scale 2^n": Value Change {
        n1640 = event-data() -> ()  [unwired: 7 out]
        n1641 = Scale By Power Of 2(n="Trap Pos. FB Out Scale 2^n", x=ext 1.0) -> (x*2^n=w2439:ext)
        n1642 = property on="Trap Pos. FB Mult Factor" class="DigNum (strict)"("Val(Sgnl)"=w2439) -> ()  [unwired: 2 in, 2 out]
      }
      event "Trap Pos FB Int Count": Value Change {
        n1643 = event-data() -> ()  [unwired: 7 out]
        n1644 = xnode "Read/Write Control"("FPGA VI Reference In"=w2442, "Trap Pos FB Int Count"="Trap Pos FB Int Count") -> ()  [unwired: 1 in, 2 out]
      }
      event "Trap pos": Value Change {
        n1645 = event-data() -> ()  [unwired: 7 out]
        n1646 = case shown="True" "Trap pos" {
          frame False {
            n1647 = property on="Trap Delta Graph" class="WFGraph (strict)"("Visible"=TRUE) -> ()  [unwired: 2 in, 2 out]
            n1648 = property on="Saved trap pos" class="WFGraph (strict)"("Visible"=FALSE) -> ()  [unwired: 2 in, 2 out]
          }
          frame True {
            n1649 = property on="Saved trap pos" class="WFGraph (strict)"("Visible"=TRUE) -> ()  [unwired: 2 in, 2 out]
            n1650 = property on="Trap Delta Graph" class="WFGraph (strict)"("Visible"=FALSE) -> ()  [unwired: 2 in, 2 out]
          }
        }
      }
    }
    "error out 2" <- w1309
    n1651 = node-c288() -> ()  [unwired: 2 out]
  }
  n1652 = timed-loop "Rough control of MCL mirror stage (debugging)" {
    tunnel: [w2451] -> w76
    timing: w22 -> [_]
    timing-out: [_] -> w21
    tunnel: w5 -> [w2449]
    stop <- w2451 stop-if-true
    n1653 = node-c288() -> ()  [unwired: 2 out]
    n1654 = case shown="2" "MCL Mode" {
      tunnel: w2449 -> [_ w2454 w2501]
      frame 0, Default {
      }
      frame 1 {
        n1655 = node-c288() -> (w2456:T23)  [unwired: 4 out]
        n1656 = timed-loop "Oscillate MCL mirror" {
          timing: w2456 -> [_]
          timing-out: [_] -> w2455
          tunnel: w2454 -> [w2457]
          i -> [w2495]
          stop <- w2458 stop-if-true
          n1657 = node-c288() -> (w2494:i64)  [unwired: 1 out]
          n1658 = Multiply(x="AO1", y=32767.0) -> (x*y=w2490:dbl)
          n1659 = Multiply(x="AO2", y=32767.0) -> (x*y=w2485:dbl)
          n1660 = Divide(x=w2490, y=10.0) -> (x/y=w2491:dbl)
          n1661 = Divide(x=w2485, y=10.0) -> (x/y=w2486:dbl)
          n1662 = To Word Integer(number=w2491) -> (16bit integer=w2483:i16)
          n1663 = To Word Integer(number=w2486) -> (16bit integer=w2482:i16)
          n1664 = Divide(x=w2494, y=i64 1000) -> (x/y=w2465:dbl)
          n1665 = Multiply(x=w2465, y=w2495) -> (x*y=w2476:dbl)
          n1666 = Multiply(x="Osc. freq. (Hz) 2", y=6.283185307179586) -> (x*y=w2477:dbl)
          n1667 = Multiply(x=w2477, y=w2476) -> (x*y=w2475:dbl)
          n1668 = Sine(x=w2475) -> (sin(x)=w2474:dbl)
          n1669 = Multiply(x=w2474, y="Osc. amp. (V)") -> (x*y=w2472:dbl)
          n1670 = Add(x=w2472, y="Osc. center (V)") -> (x+y=w2470:dbl)
          n1671 = Divide(x=w2470, y=10.0) -> (x/y=w2468:dbl)
          n1672 = Multiply(x=w2468, y=32767.0) -> (x*y=w2463:dbl)
          n1673 = Select(t=w2463, s="Scan axis", f=w2483) -> (s? t:f=w2481:dbl)
          n1674 = Select(t=w2482, s="Scan axis", f=w2463) -> (s? t:f=w2480:dbl)
          n1675 = local read "MCL Mode"() -> (w2462:u16)
          n1676 = Not Equal?(x=w2462, y=u16 1) -> (x != y?=w2459:bool)
          n1677 = local read "Stop All"() -> (w2460:bool)
          n1678 = xnode "Read/Write Control"("FPGA VI Reference In"=w2457, "AO1"=w2481, "AO2"=w2480) -> ()  [unwired: 1 in, 2 out]
          n1679 = Compound Arithmetic op=OR(w2460, w2459) -> (w2458:bool)
          n1680 = node-c288() -> ()  [unwired: 2 out]
        }
        n1681 = node-c288(w2455) -> ()  [unwired: 1 out]
      }
      frame 2 {
        n1682 = case shown="True" "Start Scan" {
          tunnel: w2501 -> [_ w2503]
          frame False {
          }
          frame True {
            n1683 = Subtract(x="End (V)", y="Begin (V)") -> (x-y=w2510:dbl)
            n1684 = Decrement(x="N Points") -> (x-1=w2509:dbl)
            n1685 = Divide(x=w2510, y=w2509) -> (x/y=w2507:dbl)
            n1686 = for {
              N: "N Points" -> [_]
              tunnel: "Begin (V)" -> [w2526]
              tunnel: [w2518] -> w2513 mode=indexing
              tunnel: w2507 -> [w2517]
              tunnel: [w2515] -> w2506 mode=indexing
              tunnel: w2503 -> [w2514]
              i -> [w2525]
              n1687 = Multiply(x=w2517, y=w2525) -> (x*y=w2524:dbl)
              n1688 = Add(x=w2526, y=w2524) -> (x+y=w2521:dbl)
              n1689 = local read "Scan axis"() -> (w2516:bool)
              n1690 = local read "AO1"() -> (w2523:dbl)
              n1691 = local read "AO2"() -> (w2522:dbl)
              n1692 = Select(t=w2521, s=w2516, f=w2523) -> (s? t:f=w2520:dbl)
              n1693 = Select(t=w2522, s=w2516, f=w2521) -> (s? t:f=w2519:dbl)
              n1694 = flat-sequence {
                tunnel: w2520 -> [w2530]
                tunnel: w2519 -> [w2529]
                tunnel: w2514 -> [w2527]
                tunnel: [w2540] -> w2518
                tunnel: [w2539] -> w2515
                frame #0 {
                  w2533 = 10.0 ("y")
                  w2528 = 32767.0 ("y")
                  n1695 = Multiply(x=w2530, y=w2528) -> (x*y=w2536:dbl)
                  n1696 = Multiply(x=w2529, y=w2528) -> (x*y=w2534:dbl)
                  n1697 = Divide(x=w2536, y=w2533) -> (x/y=w2537:dbl)
                  n1698 = Divide(x=w2534, y=w2533) -> (x/y=w2535:dbl)
                  n1699 = To Word Integer(number=w2537) -> (16bit integer=w2531:i16)
                  n1700 = To Word Integer(number=w2535) -> (16bit integer=w2532:i16)
                  n1701 = xnode "Read/Write Control"("FPGA VI Reference In"=w2527, "AO1"=w2531, "AO2"=w2532) -> ()  [unwired: 1 in, 2 out]
                }
                frame #1 {
                  n1702 = Wait (ms)(milliseconds to wait="DAQ Delay (ms)") -> ()  [unwired: 1 out]
                }
                frame #2 {
                  n1703 = local read "Slow mean"() -> (w2540:dbl)
                  n1704 = local read "Sigma"() -> (w2539:dbl)
                }
              }
            }
            n1705 = Bundle("Begin (V)"="Begin (V)", w2507, w2513) -> (→"MCL Scan":cluster{"Begin (V)":dbl, dbl, dbl[]})  [unwired: 1 out]
            n1706 = Bundle("Begin (V)"="Begin (V)", w2507, w2506) -> (→"MCL Scan 2":cluster{"Begin (V)":dbl, dbl, dbl[]})  [unwired: 1 out]
          }
        }
      }
    }
    n1707 = local read "Stop All"() -> (w2451:bool)
    n1708 = node-c288() -> ()  [unwired: 2 out]
  }
  n1709 = timed-loop "Mouse control: trap position (AOM deflection), set confocal spot from image" {
    tunnel: [w2542] -> w74
    timing: w68 -> [_]
    timing-out: [_] -> w67
    tunnel: w5 -> [w2541]
    stop <- w2542 stop-if-true
    n1710 = node-c288() -> ()  [unwired: 2 out]
    n1711 = event shown="[0] \"Pane\": Mouse Down" {
      selector: _ -> [_ _]
      dyn-events: _ -> [_ _]
      timeout: _ -> [_ _]
      tunnel: w2541 -> [w2545 _]
      event Mouse Down {
        n1712 = event-data() -> ("Time"=w2547:u32, "Coords"=w2546:T7, "Button"=w2548:u16)  [unwired: 6 out]
        n1713 = case shown="3" w2548 {
          tunnel: w2547 -> [_ _ w2654]
          tunnel: w2546 -> [_ w2585 w2652]
          tunnel: w2545 -> [_ _ w2648]
          frame 0, Default {
          }
          frame 1 {
            n1714 = property on="APD 2" class="ImageControl"() -> ("Displayed Image Position"=w2555:cluster{"Left":i32, "Top":i32})  [unwired: 2 in, 2 out]
            n1715 = property on="APD 1" class="ImageControl"() -> ("Displayed Image Position"=w2584:cluster{"Left":i32, "Top":i32})  [unwired: 2 in, 2 out]
            n1716 = property on="Detection Laser X" class="ImageControl"() -> ("Displayed Image Position"=w2581:cluster{"Left":i32, "Top":i32})  [unwired: 2 in, 2 out]
            n1717 = property on="Detection Laser Y" class="ImageControl"() -> ("Displayed Image Position"=w2580:cluster{"Left":i32, "Top":i32})  [unwired: 2 in, 2 out]
            n1718 = property on="APD 2" class="ImageControl"() -> ("Displayed Image Size"=w2554:cluster{"Width":u32, "Height":u32})  [unwired: 2 in, 2 out]
            n1719 = property on="APD 1" class="ImageControl"() -> ("Displayed Image Size"=w2582:cluster{"Width":u32, "Height":u32})  [unwired: 2 in, 2 out]
            n1720 = property on="Detection Laser X" class="ImageControl"() -> ("Displayed Image Size"=w2583:cluster{"Width":u32, "Height":u32})  [unwired: 2 in, 2 out]
            n1721 = property on="Detection Laser Y" class="ImageControl"() -> ("Displayed Image Size"=w2579:cluster{"Width":u32, "Height":u32})  [unwired: 2 in, 2 out]
            n1722 = Unbundle By Name(w2554) -> ("Width"=w2551:u32, "Height"=w2550:u32)
            n1723 = Unbundle By Name(w2555) -> ("Left"=w2553:i32, "Top"=w2552:i32)
            n1724 = Unbundle By Name(w2582) -> ("Width"=w2576:u32, "Height"=w2575:u32)
            n1725 = Unbundle By Name(w2583) -> ("Width"=w2572:u32, "Height"=w2571:u32)
            n1726 = Unbundle By Name(w2579) -> ("Width"=w2568:u32, "Height"=w2567:u32)
            n1727 = Unbundle By Name(w2584) -> ("Left"=w2578:i32, "Top"=w2577:i32)
            n1728 = Unbundle By Name(w2581) -> ("Left"=w2574:i32, "Top"=w2573:i32)
            n1729 = Unbundle By Name(w2580) -> ("Left"=w2570:i32, "Top"=w2569:i32)
            n1730 = Bundle("Left"=w2553, "Top"=w2552, "Width"=w2551, "Height"=w2550) -> (w2549:T33)  [unwired: 1 in]
            n1731 = Bundle("Left"=w2578, "Top"=w2577, "Width"=w2576, "Height"=w2575) -> (w2566:T33)  [unwired: 1 in]
            n1732 = Bundle("Left"=w2574, "Top"=w2573, "Width"=w2572, "Height"=w2571) -> (w2565:T33)  [unwired: 1 in]
            n1733 = Bundle("Left"=w2570, "Top"=w2569, "Width"=w2568, "Height"=w2567) -> (w2564:T33)  [unwired: 1 in]
            n1734 = Build Cluster Array(w2549, w2566, w2565, w2564) -> (w2563:T34)
            n1735 = for {
              tunnel: w2585 -> [w2596]
              tunnel: w2563 -> [w2597] mode=indexing
              shift-right: [w2594] -> w2561
              shift-left: TRUE -> [w2595]
              shift-right: [w2593] -> w2559
              shift-left: _ -> [w2589]
              shift-right: [w2592] -> w2558
              shift-left: _ -> [w2588]
              shift-right: [w2591] -> w2557
              shift-left: _ -> [w2587]
              shift-right: [w2590] -> w2556
              shift-left: _ -> [w2586]
              n1736 = case shown="True" w2595 {
                selector: w2595 -> [w2602 _]
                tunnel: w2597 -> [_ w2611]
                tunnel: w2596 -> [_ w2609]
                tunnel: [w2602 w2607] -> w2594
                tunnel: [w2601 w2606] -> w2593
                tunnel: [w2600 w2605] -> w2592
                tunnel: [w2599 w2604] -> w2591
                tunnel: [w2598 w2603] -> w2590
                tunnel: w2589 -> [w2601 _]
                tunnel: w2588 -> [w2600 _]
                tunnel: w2587 -> [w2599 _]
                tunnel: w2586 -> [w2598 _]
                frame False {
                }
                frame True {
                  n1737 = Unbundle(w2611) -> (w2610:T33)
                  n1738 = call "isclickinwindow.vi"("Image Param"=w2610, "Point32"=w2609) -> ("4 Y"=w2603:i32, "3 Height"=w2604:i32, "2 X"=w2605:i32, "1 Width"=w2606:i32, "In image?"=w2608:bool)  [unwired: 1 in]
                  n1739 = Not(x=w2608) -> (.not. x?=w2607:bool)
                }
              }
            }
            n1740 = Not(x=w2561) -> (.not. x?=w2560:bool)
            n1741 = case shown="True" w2560 {
              tunnel: w2558 -> [_ w2625]
              tunnel: w2556 -> [_ w2624]
              tunnel: w2559 -> [_ w2623]
              tunnel: w2557 -> [_ w2622]
              frame False {
              }
              frame True {
                w2612 = FALSE ("Get Point")
                n1742 = local read "Scan lines (y)"() -> (w2627:u64)
                n1743 = disable-structure shown="Disabled" {
                  frame Disabled {
                  }
                  frame Enabled {
                  }
                }
                n1744 = local read "Actual MCL Inc (V)"() -> (w2621:dbl)
                n1745 = local read "Scan steps (MCL)"() -> (w2626:u64)
                n1746 = Divide "Y Pix/step"(x=w2622, y=w2627) -> (x/y=w2634:dbl)
                n1747 = Divide "Y V/pix"(x=w2621, y=w2634) -> (x/y=w2633:dbl)
                n1748 = Divide "Y half step offset"(x=w2621, y=2.0) -> (x/y=w2635:dbl)